vi "Dresden R2R Sputter 03.02.2018 IY24.vi"() -> ()   [LabVIEW 2009] (continued)
                                }
                                frame #1 {
                                }
                                }
                                }
                                frame #3 {
                                n24111 = local read "Semi"() -> (w29590:bool)
                                n24112 = case shown="False" w29590 {
                                frame #0 {
                                n24113 = local read "Pc_bv_closed_ch1"() -> (w29591:bool)
                                n24114 = case shown="False" w29591 {
                                frame #0 {
                                n24115 = local write "Pc_bv1_auto_close"(TRUE ("Pc_bv1_auto_open")) -> ()
                                }
                                frame #1 {
                                }
                                }
                                }
                                frame #1 {
                                }
                                }
                                }
                                frame #4 {
                                n24116 = local read "Semi"() -> (w29593:bool)
                                n24117 = case shown="False" w29593 {
                                frame #0 {
                                n24118 = local read "Pc_bv_closed_ch1"() -> (w29594:bool)
                                n24119 = case shown="False" w29594 {
                                frame #0 {
                                n24120 = Wait (ms)(milliseconds to wait=u32 1000) -> ()  [unwired: 1 out]
                                }
                                frame #1 {
                                }
                                }
                                }
                                frame #1 {
                                }
                                }
                                }
                                frame #5 {
                                n24121 = local read "Semi"() -> (w29596:bool)
                                n24122 = case shown="False" w29596 {
                                frame #0 {
                                n24123 = while {
                                i -> [w29602]
                                stop <- w29598 stop-if-true
                                n24124 = local read "Pc_bv_closed_ch1"() -> (w29600:bool)
                                n24125 = Greater?(x=w29602, y=120) -> (0:w29601:bool)
                                n24126 = local read "Semi"() -> (w29599:bool)
                                n24127 = Compound Arithmetic op=OR(w29599, w29600, w29601) -> (w29598:bool)
                                n24128 = Wait (ms)(milliseconds to wait=u32 500) -> ()  [unwired: 1 out]
                                }
                                }
                                frame #1 {
                                }
                                }
                                }
                                frame #6 {
                                n24129 = local read "Semi"() -> (w29604:bool)
                                n24130 = case shown="False" w29604 {
                                frame #0 {
                                n24131 = local read "Pc_bv_closed_ch1"() -> (w29605:bool)
                                n24132 = case shown="False" w29605 {
                                frame #0 {
                                n24133 = local write "Error Message"("Start up process  cancelled\nbecause  PC-BV not closed.\nPlease check PC-BV1 connections." ("Error Message")) -> ()
                                n24134 = Wait (ms)(milliseconds to wait=u32 1000) -> ()  [unwired: 1 out]
                                }
                                frame #1 {
                                }
                                }
                                }
                                frame #1 {
                                }
                                }
                                }
                                }
                                }
                                frame #1 {
                                }
                                }
                                }
                                frame #1 {
                                n24135 = local read "Semi"() -> (w29608:bool)
                                n24136 = case shown="False" w29608 {
                                frame #0 {
                                n24137 = local write "SMW5"(TRUE ("CMW2")) -> ()
                                n24138 = Wait (ms)(milliseconds to wait=u32 1000) -> ()  [unwired: 1 out]
                                }
                                frame #1 {
                                }
                                }
                                }
                                }
                                }
                                frame #6 {
                                # "SOV-AR OPEN"
                                n24139 = stacked-sequence {
                                frame #0 {
                                n24140 = local read "Semi"() -> (w29611:bool)
                                n24141 = case shown="False" w29611 {
                                frame #0 {
                                n24142 = while {
                                i -> [w29617]
                                stop <- w29612 stop-if-true
                                n24143 = Greater?(x=w29617, y=50) -> (0:w29616:bool)
                                n24144 = case shown="True" w29616 {
                                frame #0 {
                                }
                                frame #1 {
                                n24145 = local write "Semi"(TRUE ("Semi")) -> ()
                                n24146 = local write "Error Message"("Coating Process  \nwas cancelled.\nPlease check \nSOV-Ar connection." ("Error Message")) -> ()
                                }
                                }
                                n24147 = local read "Ch1_Sov_Ar_di"() -> (w29615:bool)
                                n24148 = case shown="False" w29615 {
                                tunnel: [FALSE TRUE] -> w29614
                                frame #0 {
                                n24149 = local write "Ch1_Sov_Ar_do"(TRUE ("Ch1_WFC_do")) -> ()
                                n24150 = Wait Until Next ms Multiple(millisecond multiple=u32 200) -> ()  [unwired: 1 out]
                                }
                                frame #1 {
                                }
                                }
                                n24151 = local read "Semi"() -> (w29613:bool)
                                n24152 = Or(x=w29614, y=w29613) -> (x .or. y?=w29612:bool)
                                }
                                }
                                frame #1 {
                                }
                                }
                                }
                                frame #1 {
                                n24153 = local read "Semi"() -> (w29625:bool)
                                n24154 = case shown="False" w29625 {
                                frame #0 {
                                n24155 = local write "SMW6"(TRUE ("CMW2")) -> ()
                                n24156 = Wait (ms)(milliseconds to wait=u32 1000) -> ()  [unwired: 1 out]
                                }
                                frame #1 {
                                }
                                }
                                }
                                }
                                }
                                frame #7 {
                                # "CHECK CHAMBER PRESSURE"
                                n24157 = stacked-sequence {
                                frame #0 {
                                n24158 = local read "Semi"() -> (w29628:bool)
                                n24159 = case shown="False" w29628 {
                                frame #0 {
                                n24160 = while {
                                i -> [w29636]
                                stop <- w29629 stop-if-true
                                n24161 = Greater?(x=w29636, y=1500) -> (0:w29635:bool)
                                n24162 = case shown="True" w29635 {
                                frame #0 {
                                }
                                frame #1 {
                                n24163 = local write "Semi"(TRUE ("Semi")) -> ()
                                n24164 = local write "Error Message"("Coating Process cancelled.\nPlease check chamber \nconnections." ("Error Message")) -> ()
                                }
                                }
                                n24165 = local read "Ch1_pressure"() -> (w29633:dbl)
                                n24166 = Greater Or Equal?(x=w29633, y=0.15 ("CHAMBER PRESSURE")) -> (x >= y?=w29632:bool)
                                n24167 = case shown="True" w29632 {
                                tunnel: [TRUE FALSE] -> w29631
                                frame #0 {
                                }
                                frame #1 {
                                n24168 = Wait Until Next ms Multiple(millisecond multiple=u32 200) -> ()  [unwired: 1 out]
                                }
                                }
                                n24169 = local read "Semi"() -> (w29630:bool)
                                n24170 = Or(x=w29631, y=w29630) -> (x .or. y?=w29629:bool)
                                }
                                }
                                frame #1 {
                                }
                                }
                                }
                                frame #1 {
                                n24171 = local read "Semi"() -> (w29643:bool)
                                n24172 = case shown="False" w29643 {
                                frame #0 {
                                n24173 = local write "SMW8"(TRUE ("CMW2")) -> ()
                                n24174 = Wait (ms)(milliseconds to wait=u32 1000) -> ()  [unwired: 1 out]
                                }
                                frame #1 {
                                }
                                }
                                }
                                }
                                }
                                frame #8 {
                                # "PC-BV OPEN"
                                n24175 = stacked-sequence {
                                frame #0 {
                                n24176 = local read "Semi"() -> (w29646:bool)
                                n24177 = case shown="False" w29646 {
                                frame #0 {
                                n24178 = stacked-sequence {
                                frame #0 {
                                n24179 = local read "Semi"() -> (w29647:bool)
                                n24180 = case shown="False" w29647 {
                                frame #0 {
                                n24181 = local write "Pc_bv1_auto_open"(TRUE ("Tp1_auto_start")) -> ()
                                }
                                frame #1 {
                                }
                                }
                                }
                                frame #1 {
                                n24182 = local read "Semi"() -> (w29649:bool)
                                n24183 = case shown="False" w29649 {
                                frame #0 {
                                n24184 = Wait (ms)(milliseconds to wait=u32 1000) -> ()  [unwired: 1 out]
                                }
                                frame #1 {
                                }
                                }
                                }
                                frame #2 {
                                n24185 = local read "Semi"() -> (w29651:bool)
                                n24186 = case shown="False" w29651 {
                                frame #0 {
                                n24187 = while {
                                i -> [w29657]
                                stop <- w29653 stop-if-true
                                n24188 = local read "Pc_bv_opened_ch1"() -> (w29655:bool)
                                n24189 = Greater?(x=w29657, y=120) -> (0:w29656:bool)
                                n24190 = local read "Semi"() -> (w29654:bool)
                                n24191 = Compound Arithmetic op=OR(w29654, w29655, w29656) -> (w29653:bool)
                                n24192 = Wait (ms)(milliseconds to wait=u32 500) -> ()  [unwired: 1 out]
                                }
                                }
                                frame #1 {
                                }
                                }
                                }
                                frame #3 {
                                n24193 = local read "Semi"() -> (w29659:bool)
                                n24194 = case shown="False" w29659 {
                                frame #0 {
                                n24195 = local read "Pc_bv_opened_ch1"() -> (w29660:bool)
                                n24196 = case shown="False" w29660 {
                                frame #0 {
                                n24197 = local write "Pc_bv1_auto_open"(TRUE ("Pc_bv1_auto_open")) -> ()
                                }
                                frame #1 {
                                }
                                }
                                }
                                frame #1 {
                                }
                                }
                                }
                                frame #4 {
                                n24198 = local read "Semi"() -> (w29662:bool)
                                n24199 = case shown="False" w29662 {
                                frame #0 {
                                n24200 = local read "Pc_bv_opened_ch1"() -> (w29663:bool)
                                n24201 = case shown="False" w29663 {
                                frame #0 {
                                n24202 = Wait (ms)(milliseconds to wait=u32 1000) -> ()  [unwired: 1 out]
                                }
                                frame #1 {
                                }
                                }
                                }
                                frame #1 {
                                }
                                }
                                }
                                frame #5 {
                                n24203 = local read "Semi"() -> (w29665:bool)
                                n24204 = case shown="False" w29665 {
                                frame #0 {
                                n24205 = while {
                                i -> [w29671]
                                stop <- w29667 stop-if-true
                                n24206 = local read "Pc_bv_opened_ch1"() -> (w29669:bool)
                                n24207 = Greater?(x=w29671, y=120) -> (0:w29670:bool)
                                n24208 = local read "Semi"() -> (w29668:bool)
                                n24209 = Compound Arithmetic op=OR(w29668, w29669, w29670) -> (w29667:bool)
                                n24210 = Wait (ms)(milliseconds to wait=u32 500) -> ()  [unwired: 1 out]
                                }
                                }
                                frame #1 {
                                }
                                }
                                }
                                frame #6 {
                                n24211 = local read "Semi"() -> (w29673:bool)
                                n24212 = case shown="False" w29673 {
                                frame #0 {
                                n24213 = local read "Pc_bv_opened_ch1"() -> (w29674:bool)
                                n24214 = case shown="False" w29674 {
                                frame #0 {
                                n24215 = local write "Error Message"("Start up process  cancelled\nbecause  PC-BV not opened.\nPlease check PC-BV1 connections." ("Error Message")) -> ()
                                n24216 = Wait (ms)(milliseconds to wait=u32 1000) -> ()  [unwired: 1 out]
                                }
                                frame #1 {
                                }
                                }
                                }
                                frame #1 {
                                }
                                }
                                }
                                }
                                }
                                frame #1 {
                                }
                                }
                                }
                                frame #1 {
                                n24217 = local read "Semi"() -> (w29677:bool)
                                n24218 = case shown="False" w29677 {
                                frame #0 {
                                n24219 = Wait (ms)(milliseconds to wait=u32 1000) -> ()  [unwired: 1 out]
                                n24220 = local write "SMW7"(TRUE ("CMW16")) -> ()
                                }
                                frame #1 {
                                }
                                }
                                }
                                }
                                }
                                frame #9 {
                                # "PC-BV %10 OPEN"
                                n24221 = stacked-sequence {
                                frame #0 {
                                n24222 = local read "Semi"() -> (w29680:bool)
                                n24223 = case shown="False" w29680 {
                                frame #0 {
                                n24224 = stacked-sequence {
                                frame #0 {
                                n24225 = local read "Semi"() -> (w29681:bool)
                                n24226 = case shown="False" w29681 {
                                frame #0 {
                                n24227 = local write "Set_position_value"(10.0 ("Set_position_value 5")) -> ()
                                }
                                frame #1 {
                                }
                                }
                                }
                                frame #1 {
                                n24228 = local read "Semi"() -> (w29683:bool)
                                n24229 = case shown="False" w29683 {
                                frame #0 {
                                n24230 = local write "Pc_bv1_auto_set position"(TRUE ("Pc_bv1_auto_set position")) -> ()
                                }
                                frame #1 {
                                }
                                }
                                }
                                frame #2 {
                                n24231 = local read "Semi"() -> (w29685:bool)
                                n24232 = case shown="False" w29685 {
                                frame #0 {
                                n24233 = local read "Ch1_Pc_bv_middle"() -> (w29686:bool)
                                n24234 = case shown="False" w29686 {
                                frame #0 {
                                n24235 = while {
                                i -> [w29689]
                                stop <- w29688 stop-if-true
                                n24236 = Greater?(x=w29689, y=30) -> (0:w29691:bool)
                                n24237 = local read "Semi"() -> (w29687:bool)
                                n24238 = case shown="False" w29687 {
                                tunnel: [FALSE TRUE] -> w29690
                                frame #0 {
                                n24239 = Wait Until Next ms Multiple(millisecond multiple=u32 200) -> ()  [unwired: 1 out]
                                }
                                frame #1 {
                                }
                                }
                                n24240 = Or(x=w29690, y=w29691) -> (x .or. y?=w29688:bool)
                                }
                                }
                                frame #1 {
                                }
                                }
                                }
                                frame #1 {
                                }
                                }
                                }
                                frame #3 {
                                n24241 = local read "Semi"() -> (w29696:bool)
                                n24242 = case shown="False" w29696 {
                                frame #0 {
                                n24243 = local read "Ch1_Pc_bv_middle"() -> (w29697:bool)
                                n24244 = case shown="False" w29697 {
                                frame #0 {
                                n24245 = stacked-sequence {
                                frame #0 {
                                n24246 = local write "Set_position_value"(10.0 ("Set_position_value 6")) -> ()
                                }
                                frame #1 {
                                n24247 = Wait (ms)(milliseconds to wait=u32 500) -> ()  [unwired: 1 out]
                                }
                                frame #2 {
                                n24248 = local write "Pc_bv1_auto_set position"(TRUE ("Pc_bv1_auto_set position")) -> ()
                                }
                                }
                                }
                                frame #1 {
                                }
                                }
                                }
                                frame #1 {
                                }
                                }
                                }
                                frame #4 {
                                n24249 = local read "Semi"() -> (w29701:bool)
                                n24250 = case shown="False" w29701 {
                                frame #0 {
                                n24251 = local read "Ch1_Pc_bv_middle"() -> (w29702:bool)
                                n24252 = case shown="False" w29702 {
                                frame #0 {
                                n24253 = while {
                                i -> [w29705]
                                stop <- w29704 stop-if-true
                                n24254 = Greater?(x=w29705, y=30) -> (0:w29707:bool)
                                n24255 = local read "Semi"() -> (w29703:bool)
                                n24256 = case shown="False" w29703 {
                                tunnel: [FALSE TRUE] -> w29706
                                frame #0 {
                                n24257 = Wait Until Next ms Multiple(millisecond multiple=u32 200) -> ()  [unwired: 1 out]
                                }
                                frame #1 {
                                }
                                }
                                n24258 = Or(x=w29706, y=w29707) -> (x .or. y?=w29704:bool)
                                }
                                }
                                frame #1 {
                                }
                                }
                                }
                                frame #1 {
                                }
                                }
                                }
                                frame #5 {
                                n24259 = local read "Semi"() -> (w29712:bool)
                                n24260 = case shown="False" w29712 {
                                frame #0 {
                                n24261 = local read "Ch1_Pc_bv_middle"() -> (w29713:bool)
                                n24262 = case shown="False" w29713 {
                                frame #0 {
                                n24263 = local write "Semi"(TRUE ("Semi")) -> ()
                                n24264 = local write "Error Message"("Coating Process cancelled.\nPlease check PC-BV1 connections." ("Error Message")) -> ()
                                }
                                frame #1 {
                                }
                                }
                                }
                                frame #1 {
                                }
                                }
                                }
                                }
                                }
                                frame #1 {
                                }
                                }
                                }
                                frame #1 {
                                n24265 = local read "Semi"() -> (w29716:bool)
                                n24266 = case shown="False" w29716 {
                                frame #0 {
                                n24267 = local write "SMW9"(TRUE ("CMW2")) -> ()
                                n24268 = Wait (ms)(milliseconds to wait=u32 1000) -> ()  [unwired: 1 out]
                                }
                                frame #1 {
                                }
                                }
                                }
                                }
                                }
                                frame #10 {
                                # "SET AR FLOW"
                                n24269 = local read "R_Web_selection"() -> (w29719:enum32{"Web", "Other"})
                                n24270 = case shown="\"Other\"" w29719 {
                                frame #0 {
                                }
                                frame #1 {
                                n24271 = stacked-sequence {
                                frame #0 {
                                n24272 = local read "Semi"() -> (w29720:bool)
                                n24273 = case shown="False" w29720 {
                                frame #0 {
                                n24274 = stacked-sequence {
                                frame #0 {
                                n24275 = local read "Semi"() -> (w29721:bool)
                                n24276 = case shown="False" w29721 {
                                frame #0 {
                                n24277 = local write "Ar_sccm"(u16 200 ("Ar_sccm1_2")) -> ()
                                }
                                frame #1 {
                                }
                                }
                                }
                                frame #1 {
                                n24278 = local read "Semi"() -> (w29723:bool)
                                n24279 = case shown="False" w29723 {
                                frame #0 {
                                n24280 = local write "Mfc_Ar _set"(TRUE ("Mfc_Ar _1_2_set")) -> ()
                                }
                                frame #1 {
                                }
                                }
                                }
                                frame #2 {
                                n24281 = local read "Semi"() -> (w29725:bool)
                                n24282 = case shown="False" w29725 {
                                frame #0 {
                                n24283 = while {
                                i -> [w29729]
                                stop <- w29731 stop-if-true
                                n24284 = Greater?(x=w29729, y=50) -> (0:w29728:bool)
                                n24285 = local read "Semi"() -> (w29727:bool)
                                n24286 = case shown="True" w29727 {
                                tunnel: [FALSE TRUE] -> w29726
                                frame #0 {
                                n24287 = Wait Until Next ms Multiple(millisecond multiple=u32 200) -> ()  [unwired: 1 out]
                                }
                                frame #1 {
                                }
                                }
                                n24288 = Or(x=w29726, y=w29728) -> (x .or. y?=w29731:bool)
                                }
                                }
                                frame #1 {
                                }
                                }
                                }
                                frame #3 {
                                n24289 = local read "Semi"() -> (w29735:bool)
                                n24290 = case shown="False" w29735 {
                                frame #0 {
                                n24291 = local read "Ar_sccm_act 5"() -> (w29737:dbl)
                                n24292 = Greater?(x=w29737, y=1) -> (0:w29736:bool)
                                n24293 = case shown="False" w29736 {
                                frame #0 {
                                n24294 = local write "Ar_sccm"(u16 200 ("Ar_sccm1_2")) -> ()
                                }
                                frame #1 {
                                }
                                }
                                }
                                frame #1 {
                                }
                                }
                                }
                                frame #4 {
                                n24295 = local read "Semi"() -> (w29740:bool)
                                n24296 = case shown="False" w29740 {
                                frame #0 {
                                n24297 = local read "Ar_sccm_act 5"() -> (w29742:dbl)
                                n24298 = Greater?(x=w29742, y=1) -> (0:w29741:bool)
                                n24299 = case shown="False" w29741 {
                                frame #0 {
                                n24300 = while {
                                i -> [w29745]
                                stop <- w29749 stop-if-true
                                n24301 = Greater?(x=w29745, y=50) -> (0:w29744:bool)
                                n24302 = local read "Semi"() -> (w29748:bool)
                                n24303 = case shown="False" w29748 {
                                tunnel: [FALSE TRUE] -> w29747
                                frame #0 {
                                n24304 = Wait Until Next ms Multiple(millisecond multiple=u32 200) -> ()  [unwired: 1 out]
                                }
                                frame #1 {
                                }
                                }
                                n24305 = Or(x=w29747, y=w29744) -> (x .or. y?=w29749:bool)
                                }
                                }
                                frame #1 {
                                }
                                }
                                }
                                frame #1 {
                                }
                                }
                                }
                                frame #5 {
                                n24306 = local read "Semi"() -> (w29753:bool)
                                n24307 = case shown="False" w29753 {
                                frame #0 {
                                n24308 = local read "Ar_sccm_act 5"() -> (w29755:dbl)
                                n24309 = Greater?(x=w29755, y=1) -> (0:w29754:bool)
                                n24310 = case shown="False" w29754 {
                                frame #0 {
                                n24311 = local write "Semi"(TRUE ("Semi")) -> ()
                                n24312 = local write "Error Message"("Coating process cancelled.\nPlease check connections." ("Error Message")) -> ()
                                }
                                frame #1 {
                                }
                                }
                                }
                                frame #1 {
                                }
                                }
                                }
                                }
                                }
                                frame #1 {
                                }
                                }
                                }
                                frame #1 {
                                n24313 = local read "Semi"() -> (w29759:bool)
                                n24314 = case shown="False" w29759 {
                                frame #0 {
                                n24315 = Wait (ms)(milliseconds to wait=u32 1000) -> ()  [unwired: 1 out]
                                n24316 = local write "SMW11"(TRUE ("CMW2")) -> ()
                                }
                                frame #1 {
                                }
                                }
                                }
                                }
                                }
                                }
                                }
                                frame #11 {
                                # "CHECK CHAMBER PRESSURE"
                                n24317 = local read "R_Web_selection"() -> (w29762:enum32{"Web", "Other"})
                                n24318 = case shown="\"Other\"" w29762 {
                                frame #0 {
                                }
                                frame #1 {
                                n24319 = stacked-sequence {
                                frame #0 {
                                n24320 = local read "Semi"() -> (w29763:bool)
                                n24321 = case shown="False" w29763 {
                                frame #0 {
                                n24322 = while {
                                i -> [w29771]
                                stop <- w29764 stop-if-true
                                n24323 = Greater?(x=w29771, y=1500) -> (0:w29770:bool)
                                n24324 = case shown="True" w29770 {
                                frame #0 {
                                }
                                frame #1 {
                                n24325 = local write "Semi"(TRUE ("Semi")) -> ()
                                n24326 = local write "Error Message"("Coating Process cancelled.\nPlease check chamber \nconnections." ("Error Message")) -> ()
                                }
                                }
                                n24327 = local read "Ch1_pressure"() -> (w29768:dbl)
                                n24328 = Greater Or Equal?(x=w29768, y=0.05 ("CHAMBER PRESSURE 2")) -> (x >= y?=w29767:bool)
                                n24329 = case shown="False" w29767 {
                                tunnel: [FALSE TRUE] -> w29766
                                frame #0 {
                                n24330 = Wait Until Next ms Multiple(millisecond multiple=u32 200) -> ()  [unwired: 1 out]
                                }
                                frame #1 {
                                }
                                }
                                n24331 = local read "Semi"() -> (w29765:bool)
                                n24332 = Or(x=w29766, y=w29765) -> (x .or. y?=w29764:bool)
                                }
                                }
                                frame #1 {
                                }
                                }
                                }
                                frame #1 {
                                n24333 = local read "Semi"() -> (w29778:bool)
                                n24334 = case shown="False" w29778 {
                                frame #0 {
                                n24335 = local write "SMW12"(TRUE ("CMW2")) -> ()
                                n24336 = Wait (ms)(milliseconds to wait=u32 1000) -> ()  [unwired: 1 out]
                                }
                                frame #1 {
                                }
                                }
                                }
                                }
                                }
                                }
                                }
                                frame #12 {
                                # "Ignite Plasma"
                                n24337 = local read "R_Web_selection"() -> (w29781:enum32{"Web", "Other"})
                                n24338 = case shown="\"Other\"" w29781 {
                                frame #0 {
                                }
                                frame #1 {
                                n24339 = stacked-sequence {
                                frame #0 {
                                n24340 = local read "Semi"() -> (w29782:bool)
                                n24341 = case shown="False" w29782 {
                                frame #0 {
                                n24342 = stacked-sequence {
                                frame #0 {
                                n24343 = local read "Semi"() -> (w29783:bool)
                                n24344 = case shown="False" w29783 {
                                frame #0 {
                                n24345 = local read "R_Single Microwave Power"() -> (w29785:dbl)
                                n24346 = Wait (ms)(milliseconds to wait=u32 200) -> ()  [unwired: 1 out]
                                n24347 = local write "Ch1_MW1"(w29785) -> ()
                                }
                                frame #1 {
                                }
                                }
                                }
                                frame #1 {
                                n24348 = local read "Semi"() -> (w29786:bool)
                                n24349 = case shown="False" w29786 {
                                frame #0 {
                                n24350 = local write "Ch1_MW1_set"(TRUE ("Microwave Power_auto_set")) -> ()
                                }
                                frame #1 {
                                }
                                }
                                }
                                frame #2 {
                                n24351 = local read "Semi"() -> (w29788:bool)
                                n24352 = case shown="False" w29788 {
                                frame #0 {
                                n24353 = Wait (ms)(milliseconds to wait=u32 1000) -> ()  [unwired: 1 out]
                                }
                                frame #1 {
                                }
                                }
                                }
                                frame #3 {
                                n24354 = local read "Semi"() -> (w29790:bool)
                                n24355 = case shown="False" w29790 {
                                frame #0 {
                                n24356 = local read "R_Single Microwave Power"() -> (w29792:dbl)
                                n24357 = Wait (ms)(milliseconds to wait=u32 200) -> ()  [unwired: 1 out]
                                n24358 = local write "Ch1_MW2"(w29792) -> ()
                                }
                                frame #1 {
                                }
                                }
                                }
                                frame #4 {
                                n24359 = local read "Semi"() -> (w29793:bool)
                                n24360 = case shown="False" w29793 {
                                frame #0 {
                                n24361 = local write "Ch1_MW2_set"(TRUE ("MW2_Power_set")) -> ()
                                }
                                frame #1 {
                                }
                                }
                                }
                                }
                                }
                                frame #1 {
                                }
                                }
                                }
                                frame #1 {
                                n24362 = local read "Semi"() -> (w29795:bool)
                                n24363 = case shown="False" w29795 {
                                frame #0 {
                                n24364 = while {
                                i -> [w29797]
                                stop <- w29799 stop-if-true
                                n24365 = Wait Until Next ms Multiple(millisecond multiple=u32 1000) -> ()  [unwired: 1 out]
                                n24366 = local read "R_Single Microwave Time"() -> (w29798:dbl)
                                n24367 = Greater Or Equal?(x=w29797, y=w29798) -> (x >= y?=w29801:bool)
                                n24368 = Subtract(x=w29798, y=w29797) -> (x-y=→"x-y 2":dbl)
                                n24369 = local read "Semi"() -> (w29800:bool)
                                n24370 = Compound Arithmetic op=OR(w29801, w29800) -> (w29799:bool)
                                }
                                }
                                frame #1 {
                                }
                                }
                                }
                                frame #2 {
                                n24371 = local read "Semi"() -> (w29803:bool)
                                n24372 = case shown="False" w29803 {
                                frame #0 {
                                n24373 = Wait (ms)(milliseconds to wait=u32 1000) -> ()  [unwired: 1 out]
                                n24374 = local write "SMW13"(TRUE ("CMW10")) -> ()
                                }
                                frame #1 {
                                }
                                }
                                }
                                }
                                }
                                }
                                }
                                frame #13 {
                                # "encoder info  add to other web selection"
                                n24375 = local read "R_Web_selection"() -> (w29806:enum32{"Web", "Other"})
                                n24376 = case shown="\"Web\", Default" w29806 {
                                frame "Web", Default {
                                # "TC -ROLL"
                                n24377 = local read "R Single Microwave Number"() -> (w29813:dbl)
                                n24378 = local read "R Single Microwave Number"() -> (w29816:dbl)
                                n24379 = Equal?(x=w29813, y=2.0) -> (x = y?=w29807:bool)
                                n24380 = Equal?(x=w29816, y=1.0) -> (x = y?=w29808:bool)
                                n24381 = Build Array(FALSE, w29808, w29807) -> (w29811:bool[])
                                n24382 = Boolean Array To Number(Boolean array=w29811) -> (number=w29812:u32)
                                n24383 = Mantissa & Exponent(0:w29812) -> (2:w29810:dbl)  [unwired: 1 out]
                                n24384 = case shown="2" w29810 {
                                frame #0 {
                                }
                                frame #1 {
                                n24385 = local read "Semi"() -> (w29817:bool)
                                n24386 = case shown="False" w29817 {
                                frame #0 {
                                n24387 = stacked-sequence {
                                frame #0 {
                                n24388 = local read "R Maximum diameter"() -> (w29822:dbl)
                                n24389 = local read "R Web speed(cm/min)"() -> (w29820:dbl)
                                n24390 = local read "R Minimum diameter"() -> (w29823:dbl)
                                n24391 = local read "R Web thicness"() -> (w29821:dbl)
                                n24392 = local read "R _Total_length"() -> (w29818:dbl)
                                n24393 = Wait (ms)(milliseconds to wait=u32 1000) -> ()  [unwired: 1 out]
                                n24394 = local write "Max Diameter"(w29822) -> ()
                                n24395 = local write "Web Thickness"(w29821) -> ()
                                n24396 = local write "Min Diameter"(w29823) -> ()
                                n24397 = local write "Web Speed"(w29820) -> ()